vi "Dresden R2R Sputter 03.02.2018 IY24.vi"() -> ()   [LabVIEW 2009] (continued)
                          stop <- w21472 stop-if-true
                          n14975 = Greater?(x=w21471, y=50) -> (0:w21469:bool)
                          n14976 = local read "Cnt_Left_limit_di"() -> (w21475:bool)
                          n14977 = case shown="True" w21469 {
                            frame #0 {
                            }
                            frame #1 {
                              n14978 = local write "Semi"(TRUE ("Semi")) -> ()
                              n14979 = local write "Error Message"("Transfer process was\ncancelled.Please check left limit sensor." ("Error Message")) -> ()
                            }
                          }
                          n14980 = case shown="False" w21475 {
                            tunnel: [FALSE ("Ch1_pet_cool_up_do") TRUE ("Ch1_pet_cool_up_do")] -> w21474
                            frame #0 {
                              n14981 = Wait Until Next ms Multiple(millisecond multiple=u32 200) -> ()  [unwired: 1 out]
                              n14982 = local write "Cnt_Left_limit_do"(TRUE ("Ch1_pet_cool_up_do")) -> ()
                            }
                            frame #1 {
                            }
                          }
                          n14983 = local read "Semi"() -> (w21473:bool)
                          n14984 = Or(x=w21474, y=w21473) -> (x .or. y?=w21472:bool)
                        }
                      }
                      frame #1 {
                      }
                    }
                  }
                  frame #4 {
                    n14985 = local read "Semi"() -> (w21482:bool)
                    n14986 = case shown="False" w21482 {
                      frame #0 {
                        n14987 = local write "CH1_2trns_18"(TRUE ("CH1_2trns_7")) -> ()
                        n14988 = Wait (ms)(milliseconds to wait=u32 500) -> ()  [unwired: 1 out]
                      }
                      frame #1 {
                      }
                    }
                  }
                }
              }
              frame #1 {
              }
            }
          }
          frame #19 {
            n14989 = local read "Semi"() -> (w21485:bool)
            n14990 = case shown="False" w21485 {
              frame #0 {
                n14991 = local write "CH1_2trns_19"(TRUE ("CH1_2trns_18")) -> ()
                n14992 = local write "Cnt_Do_Buzzer"(TRUE ("Transfer_ch1_2")) -> ()
                n14993 = Wait (ms)(milliseconds to wait=u32 1500) -> ()  [unwired: 1 out]
              }
              frame #1 {
              }
            }
          }
          frame #20 {
            n14994 = local read "Semi"() -> (w21489:bool)
            n14995 = case shown="False" w21489 {
              frame #0 {
                n14996 = local write "ch_present_position"(3.0 ("ch_present_position")) -> ()
                n14997 = local write "Transfer_ch4_3"(FALSE ("Transfer_ch1_2")) -> ()
                n14998 = local write "Cnt_Do_Buzzer"(FALSE ("Transfer_ch1_2")) -> ()
                n14999 = Wait (ms)(milliseconds to wait=u32 500) -> ()  [unwired: 1 out]
              }
              frame #1 {
              }
            }
          }
        }
      }
    }
  }
  n15000 = while {
    stop <- FALSE stop-if-true
    n15001 = Wait Until Next ms Multiple(millisecond multiple=u32 300) -> ()  [unwired: 1 out]
    n15002 = Or(x="Set", y="Auto_set_transfer") -> (x .or. y?=w21495:bool)
    n15003 = case shown="True" w21495 {
      frame #0 {
      }
      frame #1 {
        n15004 = local read "ch_present_position"() -> (w21500:dbl)
        n15005 = local read "Set chamber"() -> (w21501:dbl)
        n15006 = Greater?(x=w21501, y=w21500) -> (0:w21499:bool)
        n15007 = case shown="True" w21499 {
          frame #0 {
            n15008 = local read "ch_present_position"() -> (w21503:dbl)
            n15009 = local read "Set chamber"() -> (w21504:dbl)
            n15010 = Subtract(x=w21504, y=w21503) -> (x-y=w21505:dbl)
            n15011 = Absolute Value(x=w21505) -> (abs(x)=w21502:dbl)
            n15012 = case shown="1" w21502 {
              frame #0 {
                n15013 = local write "final_process_messages"("Please Choose another chamber!!!" ("final_process_messages")) -> ()
              }
              frame #1 {
                n15014 = local read "ch_present_position"() -> (w21507:dbl)
                n15015 = case shown="3" w21507 {
                  frame #0 {
                  }
                  frame #1 {
                    n15016 = stacked-sequence {
                      frame #0 {
                        n15017 = local write "Transfer_ch1_2"(TRUE ("1den2")) -> ()
                        n15018 = Wait (ms)(milliseconds to wait=u32 100) -> ()  [unwired: 1 out]
                      }
                      frame #1 {
                        n15019 = while {
                          stop <- w21510 stop-if-true
                          n15020 = Wait Until Next ms Multiple(millisecond multiple=u32 300) -> ()  [unwired: 1 out]
                          n15021 = local read "Transfer_ch1_2"() -> (w21513:bool)
                          n15022 = local read "Semi"() -> (w21512:bool)
                          n15023 = Not(x=w21513) -> (.not. x?=w21511:bool)
                          n15024 = Or(x=w21512, y=w21511) -> (x .or. y?=w21510:bool)
                        }
                      }
                      frame #2 {
                        n15025 = local write "Auto_set_transfer"(FALSE ("Auto_set_transfer")) -> ()
                      }
                    }
                  }
                  frame #2 {
                    n15026 = stacked-sequence {
                      frame #0 {
                        n15027 = local write "Transfer_ch2_3"(TRUE ("1den2")) -> ()
                        n15028 = Wait (ms)(milliseconds to wait=u32 100) -> ()  [unwired: 1 out]
                      }
                      frame #1 {
                        n15029 = while {
                          stop <- w21518 stop-if-true
                          n15030 = Wait Until Next ms Multiple(millisecond multiple=u32 300) -> ()  [unwired: 1 out]
                          n15031 = local read "Transfer_ch2_3"() -> (w21521:bool)
                          n15032 = local read "Semi"() -> (w21520:bool)
                          n15033 = Not(x=w21521) -> (.not. x?=w21519:bool)
                          n15034 = Or(x=w21520, y=w21519) -> (x .or. y?=w21518:bool)
                        }
                      }
                      frame #2 {
                        n15035 = local write "Auto_set_transfer"(FALSE ("Auto_set_transfer")) -> ()
                      }
                    }
                  }
                  frame #3 {
                    n15036 = stacked-sequence {
                      frame #0 {
                        n15037 = local write "Transfer_ch3_4"(TRUE ("1den2")) -> ()
                        n15038 = Wait (ms)(milliseconds to wait=u32 100) -> ()  [unwired: 1 out]
                      }
                      frame #1 {
                        n15039 = while {
                          stop <- w21526 stop-if-true
                          n15040 = Wait Until Next ms Multiple(millisecond multiple=u32 300) -> ()  [unwired: 1 out]
                          n15041 = local read "Transfer_ch3_4"() -> (w21529:bool)
                          n15042 = local read "Semi"() -> (w21528:bool)
                          n15043 = Not(x=w21529) -> (.not. x?=w21527:bool)
                          n15044 = Or(x=w21528, y=w21527) -> (x .or. y?=w21526:bool)
                        }
                      }
                      frame #2 {
                        n15045 = local write "Auto_set_transfer"(FALSE ("Auto_set_transfer")) -> ()
                      }
                    }
                  }
                }
              }
              frame #2 {
                n15046 = local read "ch_present_position"() -> (w21532:dbl)
                n15047 = case shown="2" w21532 {
                  frame #0 {
                  }
                  frame #1 {
                    n15048 = stacked-sequence {
                      frame #0 {
                        n15049 = local write "Transfer_ch1_2"(TRUE ("1den2")) -> ()
                        n15050 = Wait (ms)(milliseconds to wait=u32 100) -> ()  [unwired: 1 out]
                      }
                      frame #1 {
                        n15051 = while {
                          stop <- w21535 stop-if-true
                          n15052 = Wait Until Next ms Multiple(millisecond multiple=u32 300) -> ()  [unwired: 1 out]
                          n15053 = local read "Transfer_ch1_2"() -> (w21538:bool)
                          n15054 = local read "Semi"() -> (w21536:bool)
                          n15055 = Not(x=w21538) -> (.not. x?=w21537:bool)
                          n15056 = Or(x=w21536, y=w21537) -> (x .or. y?=w21535:bool)
                        }
                      }
                      frame #2 {
                        n15057 = local write "Transfer_ch2_3"(TRUE ("1den2")) -> ()
                        n15058 = Wait (ms)(milliseconds to wait=u32 100) -> ()  [unwired: 1 out]
                      }
                      frame #3 {
                        n15059 = while {
                          stop <- w21542 stop-if-true
                          n15060 = Wait Until Next ms Multiple(millisecond multiple=u32 300) -> ()  [unwired: 1 out]
                          n15061 = local read "Transfer_ch2_3"() -> (w21545:bool)
                          n15062 = local read "Semi"() -> (w21544:bool)
                          n15063 = Not(x=w21545) -> (.not. x?=w21543:bool)
                          n15064 = Or(x=w21544, y=w21543) -> (x .or. y?=w21542:bool)
                        }
                      }
                      frame #4 {
                        n15065 = local write "Auto_set_transfer"(FALSE ("Auto_set_transfer")) -> ()
                      }
                    }
                  }
                  frame #2 {
                    n15066 = stacked-sequence {
                      frame #0 {
                        n15067 = local write "Transfer_ch2_3"(TRUE ("1den2")) -> ()
                        n15068 = Wait (ms)(milliseconds to wait=u32 100) -> ()  [unwired: 1 out]
                      }
                      frame #1 {
                        n15069 = while {
                          stop <- w21550 stop-if-true
                          n15070 = Wait Until Next ms Multiple(millisecond multiple=u32 300) -> ()  [unwired: 1 out]
                          n15071 = local read "Transfer_ch2_3"() -> (w21553:bool)
                          n15072 = local read "Semi"() -> (w21552:bool)
                          n15073 = Not(x=w21553) -> (.not. x?=w21551:bool)
                          n15074 = Or(x=w21552, y=w21551) -> (x .or. y?=w21550:bool)
                        }
                      }
                      frame #2 {
                        n15075 = local write "Transfer_ch3_4"(TRUE ("1den2")) -> ()
                        n15076 = Wait (ms)(milliseconds to wait=u32 100) -> ()  [unwired: 1 out]
                      }
                      frame #3 {
                        n15077 = while {
                          stop <- w21557 stop-if-true
                          n15078 = Wait Until Next ms Multiple(millisecond multiple=u32 300) -> ()  [unwired: 1 out]
                          n15079 = local read "Transfer_ch3_4"() -> (w21560:bool)
                          n15080 = local read "Semi"() -> (w21559:bool)
                          n15081 = Not(x=w21560) -> (.not. x?=w21558:bool)
                          n15082 = Or(x=w21559, y=w21558) -> (x .or. y?=w21557:bool)
                        }
                      }
                      frame #4 {
                        n15083 = local write "Auto_set_transfer"(FALSE ("Auto_set_transfer")) -> ()
                      }
                    }
                  }
                }
              }
              frame #3 {
                n15084 = local read "ch_present_position"() -> (w21563:dbl)
                n15085 = case shown="1" w21563 {
                  frame #0 {
                  }
                  frame #1 {
                    n15086 = stacked-sequence {
                      frame #0 {
                        n15087 = local write "Transfer_ch1_2"(TRUE ("1den2")) -> ()
                        n15088 = Wait (ms)(milliseconds to wait=u32 100) -> ()  [unwired: 1 out]
                      }
                      frame #1 {
                        n15089 = while {
                          stop <- w21566 stop-if-true
                          n15090 = Wait Until Next ms Multiple(millisecond multiple=u32 300) -> ()  [unwired: 1 out]
                          n15091 = local read "Transfer_ch1_2"() -> (w21569:bool)
                          n15092 = local read "Semi"() -> (w21568:bool)
                          n15093 = Not(x=w21569) -> (.not. x?=w21567:bool)
                          n15094 = Or(x=w21568, y=w21567) -> (x .or. y?=w21566:bool)
                        }
                      }
                      frame #2 {
                        n15095 = local write "Transfer_ch2_3"(TRUE ("1den2")) -> ()
                        n15096 = Wait (ms)(milliseconds to wait=u32 100) -> ()  [unwired: 1 out]
                      }
                      frame #3 {
                        n15097 = while {
                          stop <- w21573 stop-if-true
                          n15098 = Wait Until Next ms Multiple(millisecond multiple=u32 300) -> ()  [unwired: 1 out]
                          n15099 = local read "Transfer_ch2_3"() -> (w21576:bool)
                          n15100 = local read "Semi"() -> (w21575:bool)
                          n15101 = Not(x=w21576) -> (.not. x?=w21574:bool)
                          n15102 = Or(x=w21575, y=w21574) -> (x .or. y?=w21573:bool)
                        }
                      }
                      frame #4 {
                        n15103 = local write "Transfer_ch3_4"(TRUE ("1den2")) -> ()
                        n15104 = Wait (ms)(milliseconds to wait=u32 100) -> ()  [unwired: 1 out]
                      }
                      frame #5 {
                        n15105 = while {
                          stop <- w21580 stop-if-true
                          n15106 = Wait Until Next ms Multiple(millisecond multiple=u32 300) -> ()  [unwired: 1 out]
                          n15107 = local read "Transfer_ch3_4"() -> (w21583:bool)
                          n15108 = local read "Semi"() -> (w21582:bool)
                          n15109 = Not(x=w21583) -> (.not. x?=w21581:bool)
                          n15110 = Or(x=w21582, y=w21581) -> (x .or. y?=w21580:bool)
                        }
                      }
                      frame #6 {
                        n15111 = local write "Auto_set_transfer"(FALSE ("Auto_set_transfer")) -> ()
                      }
                    }
                  }
                }
              }
            }
          }
          frame #1 {
            n15112 = local read "ch_present_position"() -> (w21587:dbl)
            n15113 = local read "Set chamber"() -> (w21588:dbl)
            n15114 = Subtract(x=w21588, y=w21587) -> (x-y=w21589:dbl)
            n15115 = Absolute Value(x=w21589) -> (abs(x)=w21586:dbl)
            n15116 = case shown="3" w21586 {
              frame #0 {
              }
              frame #1 {
                n15117 = local read "ch_present_position"() -> (w21590:dbl)
                n15118 = case shown="4" w21590 {
                  frame #0 {
                  }
                  frame #1 {
                    n15119 = stacked-sequence {
                      frame #0 {
                        n15120 = local write "Transfer_ch2_1"(TRUE ("1den2")) -> ()
                        n15121 = Wait (ms)(milliseconds to wait=u32 100) -> ()  [unwired: 1 out]
                      }
                      frame #1 {
                        n15122 = while {
                          stop <- w21593 stop-if-true
                          n15123 = Wait Until Next ms Multiple(millisecond multiple=u32 300) -> ()  [unwired: 1 out]
                          n15124 = local read "Transfer_ch2_1"() -> (w21596:bool)
                          n15125 = local read "Semi"() -> (w21595:bool)
                          n15126 = Not(x=w21596) -> (.not. x?=w21594:bool)
                          n15127 = Or(x=w21595, y=w21594) -> (x .or. y?=w21593:bool)
                        }
                      }
                      frame #2 {
                        n15128 = local write "Auto_set_transfer"(FALSE ("Auto_set_transfer")) -> ()
                      }
                    }
                  }
                  frame #2 {
                    n15129 = stacked-sequence {
                      frame #0 {
                        n15130 = local write "Transfer_ch3_2"(TRUE ("1den2")) -> ()
                        n15131 = Wait (ms)(milliseconds to wait=u32 100) -> ()  [unwired: 1 out]
                      }
                      frame #1 {
                        n15132 = while {
                          stop <- w21601 stop-if-true
                          n15133 = Wait Until Next ms Multiple(millisecond multiple=u32 300) -> ()  [unwired: 1 out]
                          n15134 = local read "Transfer_ch3_2"() -> (w21604:bool)
                          n15135 = local read "Semi"() -> (w21603:bool)
                          n15136 = Not(x=w21604) -> (.not. x?=w21602:bool)
                          n15137 = Or(x=w21603, y=w21602) -> (x .or. y?=w21601:bool)
                        }
                      }
                      frame #2 {
                        n15138 = local write "Auto_set_transfer"(FALSE ("Auto_set_transfer")) -> ()
                      }
                    }
                  }
                  frame #3 {
                    n15139 = stacked-sequence {
                      frame #0 {
                        n15140 = local write "Transfer_ch4_3"(TRUE ("1den2")) -> ()
                        n15141 = Wait (ms)(milliseconds to wait=u32 100) -> ()  [unwired: 1 out]
                      }
                      frame #1 {
                        n15142 = while {
                          stop <- w21609 stop-if-true
                          n15143 = Wait Until Next ms Multiple(millisecond multiple=u32 300) -> ()  [unwired: 1 out]
                          n15144 = local read "Transfer_ch4_3"() -> (w21612:bool)
                          n15145 = local read "Semi"() -> (w21611:bool)
                          n15146 = Not(x=w21612) -> (.not. x?=w21610:bool)
                          n15147 = Or(x=w21611, y=w21610) -> (x .or. y?=w21609:bool)
                        }
                      }
                      frame #2 {
                        n15148 = local write "Auto_set_transfer"(FALSE ("Auto_set_transfer")) -> ()
                      }
                    }
                  }
                }
              }
              frame #2 {
                n15149 = local read "ch_present_position"() -> (w21615:dbl)
                n15150 = case shown="4" w21615 {
                  frame #0 {
                  }
                  frame #1 {
                    n15151 = stacked-sequence {
                      frame #0 {
                        n15152 = local write "Transfer_ch3_2"(TRUE ("1den2")) -> ()
                        n15153 = Wait (ms)(milliseconds to wait=u32 100) -> ()  [unwired: 1 out]
                      }
                      frame #1 {
                        n15154 = while {
                          stop <- w21618 stop-if-true
                          n15155 = Wait Until Next ms Multiple(millisecond multiple=u32 300) -> ()  [unwired: 1 out]
                          n15156 = local read "Transfer_ch3_2"() -> (w21621:bool)
                          n15157 = local read "Semi"() -> (w21620:bool)
                          n15158 = Not(x=w21621) -> (.not. x?=w21619:bool)
                          n15159 = Or(x=w21620, y=w21619) -> (x .or. y?=w21618:bool)
                        }
                      }
                      frame #2 {
                        n15160 = local write "Transfer_ch2_1"(TRUE ("1den2")) -> ()
                        n15161 = Wait (ms)(milliseconds to wait=u32 100) -> ()  [unwired: 1 out]
                      }
                      frame #3 {
                        n15162 = while {
                          stop <- w21625 stop-if-true
                          n15163 = Wait Until Next ms Multiple(millisecond multiple=u32 300) -> ()  [unwired: 1 out]
                          n15164 = local read "Transfer_ch2_1"() -> (w21628:bool)
                          n15165 = local read "Semi"() -> (w21627:bool)
                          n15166 = Not(x=w21628) -> (.not. x?=w21626:bool)
                          n15167 = Or(x=w21627, y=w21626) -> (x .or. y?=w21625:bool)
                        }
                      }
                      frame #4 {
                        n15168 = local write "Auto_set_transfer"(FALSE ("Auto_set_transfer")) -> ()
                      }
                    }
                  }
                  frame #2 {
                    n15169 = stacked-sequence {
                      frame #0 {
                        n15170 = local write "Transfer_ch4_3"(TRUE ("1den2")) -> ()
                        n15171 = Wait (ms)(milliseconds to wait=u32 100) -> ()  [unwired: 1 out]
                      }
                      frame #1 {
                        n15172 = while {
                          stop <- w21633 stop-if-true
                          n15173 = Wait Until Next ms Multiple(millisecond multiple=u32 300) -> ()  [unwired: 1 out]
                          n15174 = local read "Transfer_ch4_3"() -> (w21636:bool)
                          n15175 = local read "Semi"() -> (w21635:bool)
                          n15176 = Not(x=w21636) -> (.not. x?=w21634:bool)
                          n15177 = Or(x=w21635, y=w21634) -> (x .or. y?=w21633:bool)
                        }
                      }
                      frame #2 {
                        n15178 = local write "Transfer_ch3_2"(TRUE ("1den2")) -> ()
                        n15179 = Wait (ms)(milliseconds to wait=u32 100) -> ()  [unwired: 1 out]
                      }
                      frame #3 {
                        n15180 = while {
                          stop <- w21640 stop-if-true
                          n15181 = Wait Until Next ms Multiple(millisecond multiple=u32 300) -> ()  [unwired: 1 out]
                          n15182 = local read "Transfer_ch3_2"() -> (w21641:bool)
                          n15183 = Not(x=w21641) -> (.not. x?=w21640:bool)
                        }
                      }
                      frame #4 {
                        n15184 = local write "Auto_set_transfer"(FALSE ("Auto_set_transfer")) -> ()
                      }
                    }
                  }
                }
              }
              frame #3 {
                n15185 = local read "ch_present_position"() -> (w21644:dbl)
                n15186 = case shown="4" w21644 {
                  frame #0 {
                  }
                  frame #1 {
                    n15187 = stacked-sequence {
                      frame #0 {
                        n15188 = local write "Transfer_ch4_3"(TRUE ("1den2")) -> ()
                        n15189 = Wait (ms)(milliseconds to wait=u32 100) -> ()  [unwired: 1 out]
                      }
                      frame #1 {
                        n15190 = while {
                          stop <- w21647 stop-if-true
                          n15191 = Wait Until Next ms Multiple(millisecond multiple=u32 300) -> ()  [unwired: 1 out]
                          n15192 = local read "Transfer_ch4_3"() -> (w21650:bool)
                          n15193 = local read "Semi"() -> (w21649:bool)
                          n15194 = Not(x=w21650) -> (.not. x?=w21648:bool)
                          n15195 = Or(x=w21649, y=w21648) -> (x .or. y?=w21647:bool)
                        }
                      }
                      frame #2 {
                        n15196 = local write "Transfer_ch3_2"(TRUE ("1den2")) -> ()
                        n15197 = Wait (ms)(milliseconds to wait=u32 100) -> ()  [unwired: 1 out]
                      }
                      frame #3 {
                        n15198 = while {
                          stop <- w21654 stop-if-true
                          n15199 = Wait Until Next ms Multiple(millisecond multiple=u32 300) -> ()  [unwired: 1 out]
                          n15200 = local read "Transfer_ch3_2"() -> (w21657:bool)
                          n15201 = local read "Semi"() -> (w21656:bool)
                          n15202 = Not(x=w21657) -> (.not. x?=w21655:bool)
                          n15203 = Or(x=w21656, y=w21655) -> (x .or. y?=w21654:bool)
                        }
                      }
                      frame #4 {
                        n15204 = local write "Transfer_ch2_1"(TRUE ("1den2")) -> ()
                        n15205 = Wait (ms)(milliseconds to wait=u32 100) -> ()  [unwired: 1 out]
                      }
                      frame #5 {
                        n15206 = while {
                          stop <- w21661 stop-if-true
                          n15207 = Wait Until Next ms Multiple(millisecond multiple=u32 300) -> ()  [unwired: 1 out]
                          n15208 = local read "Transfer_ch2_1"() -> (w21664:bool)
                          n15209 = local read "Semi"() -> (w21663:bool)
                          n15210 = Not(x=w21664) -> (.not. x?=w21662:bool)
                          n15211 = Or(x=w21663, y=w21662) -> (x .or. y?=w21661:bool)
                        }
                      }
                      frame #6 {
                        n15212 = local write "Auto_set_transfer"(FALSE ("Auto_set_transfer")) -> ()
                      }
                    }
                  }
                }
              }
            }
          }
        }
      }
    }
  }
  n15213 = while {
    stop <- i16? 0 stop-if-true
    n15214 = case shown="True" "Start_up_ch1" {
      frame #0 {
      }
      frame #1 {
        # "START UP OF CH1 PROCEDURE"
        n15215 = stacked-sequence {
          frame #0 {
            # "ROUTINE CHECK"
            n15216 = local read "Semi"() -> (w27244:bool)
            n15217 = case shown="False" w27244 {
              frame #0 {
                n15218 = stacked-sequence {
                  frame #0 {
                    n15219 = local write "Clean_Pumping_ch1"(TRUE) -> ()
                    n15220 = local write "final_process_messages"("Start up process was completed." ("final_process_messages")) -> ()
                    n15221 = local write "system_status"("Start up process continues." ("system_status")) -> ()
                    n15222 = property on="Pressure_time_graph_ch1" class="WFChart (strict)"("History Data"=dbl[] []) -> ()  [unwired: 2 in, 2 out]
                    n15223 = Wait (ms)(milliseconds to wait=u32 1000) -> ()  [unwired: 1 out]
                  }
                  frame #1 {
                    n15224 = local read "Semi"() -> (w27250:bool)
                    n15225 = case shown="False" w27250 {
                      frame #0 {
                        n15226 = stacked-sequence {
                          frame #0 {
                            n15227 = local read "Semi"() -> (w27251:bool)
                            n15228 = case shown="False" w27251 {
                              frame #0 {
                                n15229 = while {
                                i -> [w27258]
                                stop <- w27254 stop-if-true
                                n15230 = Greater?(x=w27258, y=50) -> (0:w27252:bool)
                                n15231 = case shown="True" w27252 {
                                frame #0 {
                                }
                                frame #1 {
                                n15232 = local write "Error Message"("Start up process cancelled because\nthere is no enough air pressure.\nPlease check air pressure connections." ("Error Message")) -> ()
                                n15233 = local write "Semi"(TRUE ("Semi")) -> ()
                                }
                                }
                                n15234 = local read "Ch1_Air_press_di"() -> (w27253:bool)
                                n15235 = case shown="True" w27253 {
                                tunnel: [TRUE FALSE] -> w27256
                                frame #0 {
                                }
                                frame #1 {
                                n15236 = Wait Until Next ms Multiple(millisecond multiple=u32 200) -> ()  [unwired: 1 out]
                                }
                                }
                                n15237 = local read "Semi"() -> (w27255:bool)
                                n15238 = Or(x=w27256, y=w27255) -> (x .or. y?=w27254:bool)
                                }
                              }
                              frame #1 {
                              }
                            }
                          }
                          frame #1 {
                            n15239 = local read "Semi"() -> (w27264:bool)
                            n15240 = case shown="False" w27264 {
                              frame #0 {
                                n15241 = Wait Until Next ms Multiple(millisecond multiple=u32 1000) -> ()  [unwired: 1 out]
                                n15242 = local write "Ch1_PA1"(TRUE ("PA0")) -> ()
                                n15243 = local write "Ch1_PV1"(TRUE ("PA0")) -> ()
                              }
                              frame #1 {
                              }
                            }
                          }
                        }
                      }
                      frame #1 {
                      }
                    }
                  }
                  frame #2 {
                    n15244 = local read "Semi"() -> (w27268:bool)
                    n15245 = case shown="False" w27268 {
                      frame #0 {
                        n15246 = stacked-sequence {
                          frame #0 {
                            n15247 = local read "Semi"() -> (w27269:bool)
                            n15248 = case shown="False" w27269 {
                              frame #0 {
                                n15249 = while {
                                i -> [w27276]
                                stop <- w27272 stop-if-true
                                n15250 = Greater?(x=w27276, y=50) -> (0:w27270:bool)
                                n15251 = case shown="True" w27270 {
                                frame #0 {
                                }
                                frame #1 {
                                n15252 = local write "Error Message"("Start up process cancelled because\nchamber door is open.\nPlease close the door." ("Error Message")) -> ()
                                n15253 = local write "Semi"(TRUE ("Semi")) -> ()
                                }
                                }
                                n15254 = local read "Ch1_Ds_di"() -> (w27271:bool)
                                n15255 = case shown="True" w27271 {
                                tunnel: [TRUE FALSE] -> w27274
                                frame #0 {
                                }
                                frame #1 {
                                n15256 = Wait Until Next ms Multiple(millisecond multiple=u32 200) -> ()  [unwired: 1 out]
                                }
                                }
                                n15257 = local read "Semi"() -> (w27273:bool)
                                n15258 = Or(x=w27274, y=w27273) -> (x .or. y?=w27272:bool)
                                }
                              }
                              frame #1 {
                              }
                            }
                          }
                          frame #1 {
                            n15259 = local read "Semi"() -> (w27282:bool)
                            n15260 = case shown="False" w27282 {
                              frame #0 {
                                n15261 = local write "Ch1_PV2"(TRUE ("PA0")) -> ()
                                n15262 = local write "Ch1_PA2"(TRUE ("PA0")) -> ()
                                n15263 = Wait Until Next ms Multiple(millisecond multiple=u32 1000) -> ()  [unwired: 1 out]
                              }
                              frame #1 {
                              }
                            }
                          }
                        }
                      }
                      frame #1 {
                      }
                    }
                  }
                  frame #3 {
                    n15264 = local read "Semi"() -> (w27286:bool)
                    n15265 = case shown="False" w27286 {
                      frame #0 {
                        n15266 = stacked-sequence {
                          frame #0 {
                            n15267 = local read "Semi"() -> (w27287:bool)
                            n15268 = case shown="False" w27287 {
                              frame #0 {
                                n15269 = while {
                                i -> [w27294]
                                stop <- w27290 stop-if-true
                                n15270 = Greater?(x=w27294, y=50) -> (0:w27288:bool)
                                n15271 = case shown="True" w27288 {
                                frame #0 {
                                }
                                frame #1 {
                                n15272 = local write "Error Message"("Start up process cancelled because\nsystem water flow is not enough.\nPlease check main water flow connections." ("Error Message")) -> ()
                                n15273 = local write "Semi"(TRUE ("Semi")) -> ()
                                }
                                }
                                n15274 = local read "Cnt_wfs_di"() -> (w27289:bool)
                                n15275 = case shown="False" w27289 {
                                tunnel: [TRUE FALSE] -> w27292
                                frame #0 {
                                }
                                frame #1 {
                                n15276 = Wait Until Next ms Multiple(millisecond multiple=u32 200) -> ()  [unwired: 1 out]
                                }
                                }
                                n15277 = local read "Semi"() -> (w27291:bool)
                                n15278 = Or(x=w27292, y=w27291) -> (x .or. y?=w27290:bool)
                                }
                              }
                              frame #1 {
                              }
                            }
                          }
                          frame #1 {
                            n15279 = local read "Semi"() -> (w27300:bool)
                            n15280 = case shown="False" w27300 {
                              frame #0 {
                                n15281 = Wait Until Next ms Multiple(millisecond multiple=u32 1000) -> ()  [unwired: 1 out]
                                n15282 = local write "Ch1_PV3"(TRUE ("PA0")) -> ()
                                n15283 = local write "Ch1_PA3"(TRUE ("PA0")) -> ()
                              }
                              frame #1 {
                              }
                            }
                          }
                        }
                      }
                      frame #1 {
                      }
                    }
                  }
                  frame #4 {
                    n15284 = local read "Semi"() -> (w27304:bool)
                    n15285 = case shown="False" w27304 {
                      frame #0 {
                        n15286 = disable-structure shown="Disabled" {
                          frame #0 {
                            n15287 = stacked-sequence {
                              frame #0 {
                                n15288 = local read "Semi"() -> (w27305:bool)
                                n15289 = case shown="False" w27305 {
                                frame #0 {
                                n15290 = local write "Ch1_WFC_do"(TRUE ("Ch1_WFC_do")) -> ()
                                }
                                frame #1 {
                                }
                                }
                              }
                              frame #1 {
                                n15291 = local read "Semi"() -> (w27307:bool)
                                n15292 = case shown="False" w27307 {
                                frame #0 {
                                n15293 = while {
                                i -> [w27314]
                                stop <- w27310 stop-if-true
                                n15294 = Greater?(x=w27314, y=50) -> (0:w27308:bool)
                                n15295 = case shown="True" w27308 {
                                frame #0 {
                                }
                                frame #1 {
                                n15296 = local write "Error Message"("Start up process cancelled because\nchamber water flow is not enough.\nPlease check chamber water \nflow connections." ("Error Message")) -> ()
                                n15297 = local write "Semi"(TRUE ("Semi")) -> ()
                                }
                                }
                                n15298 = local read "Ch1_WFS_di"() -> (w27309:bool)
                                n15299 = case shown="False" w27309 {
                                tunnel: [TRUE FALSE] -> w27312
                                frame #0 {
                                }
                                frame #1 {
                                n15300 = Wait Until Next ms Multiple(millisecond multiple=u32 200) -> ()  [unwired: 1 out]
                                n15301 = local write "Ch1_WFC_do"(TRUE ("Ch1_WFC_do")) -> ()
                                }
                                }
                                n15302 = local read "Semi"() -> (w27311:bool)
                                n15303 = Or(x=w27312, y=w27311) -> (x .or. y?=w27310:bool)
                                }
                                }
                                frame #1 {
                                }
                                }
                              }
                              frame #2 {
                                n15304 = local read "Semi"() -> (w27321:bool)
                                n15305 = case shown="False" w27321 {
                                frame #0 {
                                n15306 = Wait Until Next ms Multiple(millisecond multiple=u32 1000) -> ()  [unwired: 1 out]
                                }
                                frame #1 {
                                }
                                }
                              }
                            }
                          }
                          frame #1 {
                          }
                        }
                      }
                      frame #1 {
                      }
                    }
                  }
                  frame #5 {
                    n15307 = local read "Semi"() -> (w27323:bool)
                    n15308 = case shown="False" w27323 {
                      frame #0 {
                        n15309 = stacked-sequence {
                          frame #0 {
                            n15310 = local read "Semi"() -> (w27324:bool)
                            n15311 = case shown="False" w27324 {
                              frame #0 {
                                n15312 = local write "Ch1_Trns_gv_close_do"(TRUE ("Ch1_WFC_do")) -> ()
                              }
                              frame #1 {
                              }
                            }
                          }
                          frame #1 {
                            n15313 = local read "Semi"() -> (w27326:bool)
                            n15314 = case shown="False" w27326 {
                              frame #0 {
                                n15315 = while {
                                i -> [w27333]
                                stop <- w27329 stop-if-true
                                n15316 = Greater?(x=w27333, y=300) -> (0:w27327:bool)
                                n15317 = case shown="True" w27327 {
                                frame #0 {
                                }
                                frame #1 {
                                n15318 = local write "Error Message"("Start up process cancelled because\nchamber Trns GV between \nCH1 and CH2 not closed.\nPlease check  GV connection." ("Error Message")) -> ()
                                n15319 = local write "Semi"(TRUE ("Semi")) -> ()
                                }
                                }
                                n15320 = local read "Ch1_Trns_gv_close_di"() -> (w27328:bool)
                                n15321 = case shown="False" w27328 {
                                tunnel: [TRUE FALSE] -> w27331
                                frame #0 {
                                }
                                frame #1 {
                                n15322 = Wait Until Next ms Multiple(millisecond multiple=u32 200) -> ()  [unwired: 1 out]
                                n15323 = local write "Ch1_Trns_gv_open_do"(FALSE ("Ch1_Trns_gv_open_do")) -> ()
                                n15324 = local write "Ch1_Trns_gv_close_do"(TRUE ("Ch1_Trns_gv_close_do")) -> ()
                                }
                                }
                                n15325 = local read "Semi"() -> (w27330:bool)
                                n15326 = Or(x=w27331, y=w27330) -> (x .or. y?=w27329:bool)
                                }
                              }
                              frame #1 {
                              }
                            }
                          }
                          frame #2 {
                            n15327 = local read "Semi"() -> (w27341:bool)
                            n15328 = case shown="False" w27341 {
                              frame #0 {
                                n15329 = Wait Until Next ms Multiple(millisecond multiple=u32 1000) -> ()  [unwired: 1 out]
                                n15330 = local write "Ch1_PV5"(TRUE ("PA0")) -> ()
                                n15331 = local write "Ch1_PA5"(TRUE ("PA0")) -> ()
                              }
                              frame #1 {
                              }
                            }
                          }
                        }
                      }
                      frame #1 {
                      }
                    }
                  }
                }
              }
              frame #1 {
              }
            }
          }
          frame #1 {
            # "ROUTINE CHECK"
            n15332 = local read "Semi"() -> (w27345)
            n15333 = case shown="False" w27345 {
              frame #0 {
                n15334 = local read "Ch1_pressure 2"() -> (w27347)
                n15335 = Greater Or Equal?(x=w27347, y=dbl? 0.9) -> (x >= y?=w27346)
                n15336 = case shown="True" w27346 {
                  frame #0 {
                    # "PUMPING CH1 LOWER THAN 0.9 TORR"
                    n15337 = local read "Semi"() -> (w27349)
                    n15338 = case shown="False" w27349 {
                      frame #0 {
                        n15339 = stacked-sequence {
                          frame #0 {
                            # "Close CH1-VBV"
                            n15340 = local read "Semi"() -> (w27350:bool)
                            n15341 = case shown="False" w27350 {
                              frame #0 {
                                n15342 = stacked-sequence {
                                frame #0 {
                                n15343 = local read "Semi"() -> (w27351:bool)
                                n15344 = case shown="False" w27351 {
                                frame #0 {
                                n15345 = while {
                                i -> [w27358]
                                stop <- w27352 stop-if-true
                                n15346 = Greater?(x=w27358, y=50) -> (0:w27356:bool)
                                n15347 = case shown="True" w27356 {